vi "IMAQdx_AbsImage_Flea3_v4.2.vi"() -> ()   [LabVIEW 2012]
doc: "Take a single PixelFly exposure and display the result as an intensity graph.This VI illustrates the basics of taking an exposure with the PixelFly camera. Use Ctrl-H to get help on any of the controls\n\nCopyright 2001, The Cooke Corporation."
uses:
  LabVIEW Data V4.10/Shared Libraries/Controls/FileName_Cluster.ctl
  <vilib>/userdefined/High Color/IMAQdx.ctl
  <vilib>/vision/driver/IMAQdx.llb/IMAQdx Acquisition Mode.ctl
  Shared Libraries/Controls/FileInfo_Global.vi
  <vilib>/Analysis/NI_AALBase.lvlib
  <vilib>/vision/driver/NI_Vision_Acquisition_Software.lvlib
panel:
  in  "Interrupt":bool
  out "Buffer Number":u32=4294967294
  out "Frames":i32
  out "Loop":i32=1
  out "Status":string="Running..."
  in  "stop":bool
  in  "Tab Control":enum32{"Setup", "Images", "Hardware status"}(tab)
  in  "Experiment":T1(ring)=enum."Sr"
  in  "Accept parameters from remote system":bool=TRUE
  in  "Bias (Amps)":dbl
  in  "Pinch Coil (Amps)":dbl=520.0
  in  "Expansion time (ms)":dbl=19.0
  in  "Trap min at 0 (MHz)":dbl=2.85
  in  "Detuning (Linewidths)":dbl
  in  "Racetrack (Amps)":dbl=540.0
  in  "Magnification":dbl=0.395
  in  "Image direction":enum16{"XY", "XZ"}(ring)=enum."XZ"
  in  "Imaging technique":enum16{"Absorption", "Fluorescence", "RawImage"}(ring)
  in  "File Parameters":T2={"Data Root"=path "C:/Experiment/Data", "Index"=8, "Instrument"="Flea3_20S4M"} {"Index" format="%04d"}
  in  "Send data to Igor?":bool=TRUE
  out "Command to Igor":string="AutoRunV3(\"MOT_test\",\"C:\\\\Experiment\\\\Data\\\\2012\\\\December\\\\06\\\\Flea3_20S4M_06Dec2012_0007.ibw\") "
  out "Image note":string="Experiment=Sr\nCamera_ID=Flea3\nImageType=Raw\nDataType=Absorption\nImageDirection=XZ\nMagnification=3.950000E-1\nFileNumber=7\n# Current Variables\n# \nplus_zman=-1.791000E+0\nminus_zman=-1.440000E+0\ncompensation=-1.536000E+0\nXshim=1.000000E+1\nYshim=0.000000E+0\nZshim=7.500000E+0\nProbePow=1.200000E+0\ntau=0.000000E+0\ntEnd=0.000000E+0\nDipStart=0.000000E+0\nMOTcurrent=-1.250000E+0\nProbeDet=0.000000E+0\nTOF=5.000000E-4\n# Master Staging List\n# Line\tMarker\tOption\tHalt\t0       4       8      12      16      20    AO\tDelay\t\tPoints\t0\t\t1\t\t2\t\t3\t\t4\t\t5\t\t6\t\t7\t\t8\t\t9\t\t10\t\t11\t\t12\t\t13\t\t14\t\t15\t\tComment\n00\t\tRamp\t0 0 0 0 0 0 0 0 0 0 0 0 1 1 1 1 0 0 0 0 0 0 0 0\t5\t0\tplus_zman\tminus_zman\tcompensation\tMOTcurrent\t0\t0\t0\t0\t0\t0\tProbePow\t0\tXshim\tYshim\tZshim\t0\tblue MOT load\n01\t\tRamp\t0 0 0 0 0 0 0 0 0 0 0 0 1 1 1 1 0 0 0 0 0 0 0 0\t.001\t0\tplus_zman\tminus_zman\tcompensation\tMOTcurrent\t0\t0\t0\t0\t0\t0\tProbePow\t0\tXshim\tYshim\tZshim\t0\tHold\n02\t\tRamp\t0 0 0 0 0 0 0 0 0 0 0 0 1 0 1 1 0 0 0 0 0 0 0 0\t.003\t0\tplus_zman\tminus_zman\tcompensation\tMOTcurrent\t0\t0\t0\t0\t0\t0\tProbePow\t0\tXshim\tYshim\tZshim\t0\tHold\n03\t\tRamp\t0 0 0 0 0 0 0 0 0 0 0 0 1 0 0 0 0 0 0 0 0 0 0 0\tTOF\t0\tplus_zman\tminus_zman\tcompensation\tMOTcurrent\t0\t0\t0\t0\t0\t0\tProbePow\t0\tXshim\tYshim\tZshim\t0\tTOF\n04\t\tRamp\t0 0 0 0 0 0 0 0 0 0 0 0 1 0 0 0 0 0 0 0 0 0 0 0\t.00002\t0\tplus_zman\tminus_zman\tcompensation\tMOTcurrent\t0\t0\t0\t0\t0\t0\tProbePow\t0\tXshim\tYshim\tZshim\t0\tatom img\n05\t\tRamp\t0 0 0 0 0 0 0 0 0 0 0 0 1 1 0 0 0 0 0 0 0 0 0 0\t.0001\t0\tplus_zman\tminus_zman\tcompensation\tMOTcurrent\t0\t0\t0\t0\t0\t0\tProbePow\t0\tXshim\tYshim\tZshim\t0\tatom img\n06\t\tRamp\t0 0 0 0 0 0 0 0 0 0 0 0 1 0 0 0 0 0 0 0 0 0 0 0\t1\t0\tplus_zman\tminus_zman\tcompensation\tMOTcurrent\t0\t0\t0\t0\t0\t0\tProbePow\t0\tXshim\tYshim\tZshim\t0\ttransmit img\n07\t\tRamp\t0 0 0 0 0 0 0 0 0 0 0 0 1 0 0 0 0 0 0 0 0 0 0 0\t.00002\t0\tplus_zman\tminus_zman\tcompensation\tMOTcurrent\t0\t0\t0\t0\t0\t0\tProbePow\t0\tXshim\tYshim\tZshim\t0\tprobe img\n08\t\tRamp\t0 0 0 0 0 0 0 0 0 0 0 0 1 1 0 0 0 0 0 0 0 0 0 0\t.0001\t0\tplus_zman\tminus_zman\tcompensation\tMOTcurrent\t0\t0\t0\t0\t0\t0\tProbePow\t0\tXshim\tYshim\tZshim\t0\tprobe img\n09\t\tRamp\t0 0 0 0 0 0 0 0 0 0 0 0 1 0 0 0 0 0 0 0 0 0 0 0\t0.5\t0\tplus_zman\tminus_zman\tcompensation\tMOTcurrent\t0\t0\t0\t0\t0\t0\tProbePow\t0\tXshim\tYshim\tZshim\t0\ttransmit img\n10\t\tRamp\t0 0 0 0 0 0 0 0 0 0 0 0 1 0 0 0 0 0 0 0 0 0 0 0\t0.5\t0\tplus_zman\tminus_zman\tcompensation\tMOTcurrent\t0\t0\t0\t0\t0\t0\tProbePow\t0\tXshim\tYshim\tZshim\t0\ttransmit img\n11\t\tRamp\t0 0 0 0 0 0 0 0 0 0 0 0 1 0 0 0 0 0 0 0 0 0 0 0\t.00012\t0\tplus_zman\tminus_zman\tcompensation\tMOTcurrent\t0\t0\t0\t0\t0\t0\tProbePow\t0\tXshim\tYshim\tZshim\t0\tbg img\n12\t\tRamp\t0 0 0 0 0 0 0 0 0 0 0 0 1 0 0 0 0 0 0 0 0 0 0 0\t1\t0\tplus_zman\tminus_zman\tcompensation\tMOTcurrent\t0\t0\t0\t0\t0\t0\tProbePow\t0\tXshim\tYshim\tZshim\t0\ttransmit img\n13\t\tRamp\t0 0 0 0 0 0 0 0 0 0 0 0 1 1 1 1 0 0 0 0 0 0 0 0\t.5\t0\tplus_zman\tminus_zman\tcompensation\tMOTcurrent\t0\t0\t0\t0\t0\t0\tProbePow\t0\tXshim\tYshim\tZshim\t0\treset\n14\t\t\t0 0 0 0 0 0 0 0 0 0 0 0 1 1 1 1 0 0 0 0 0 0 0 0\t.1\t0\t\t\t\t\t\t\t\t\t\t\t\t\t\t\t\t\treset\n# Slave Staging List\n# Line\tMarker\tOption\tHalt\t0       4       8      12      16      20    AO\tDelay\t\tPoints\t0\t\t1\t\t2\t\t3\t\t4\t\t5\t\t6\t\t7\t\t8\t\t9\t\t10\t\t11\t\t12\t\t13\t\t14\t\t15\t\tComment\n# SRS List\n# \n#\n# Evaporation\n\nDDS Table\r\n"
  in  "Igor Wave Name":string="Test_Img"
  in  "Save file to archive?":bool=TRUE
  in  "Timeout (ms)":u32=1500
  in  "Gain":dbl
  in  "Shutter speed":dbl=0.03
  in  "Camera Name":T3="Abs XZ"
  out "Timeout":bool=TRUE
  out "Trigger Overrun":bool=TRUE
  in  "Quad [Amps]":dbl=540.0
  in  "Source of File Data":refnum<k21>="\\\\Control\\VariableLibrary\\Instruction String"
  in  "Bits to shift":i32
  in  "Raw image to view":u16(ring) items=["Absorbtion", "Probe", "Background"]
  in  "Update Graphics":bool=TRUE
  out "Raw Image":u16[][](graph)
  out "Processed Image":sgl[][](graph)
  out "Histogram":cluster{"X Values":dbl[], dbl[]}(graph)={"X Values"=[0.296875, 0.890625, 1.484375, 2.078125, 2.671875, 3.265625, 3.859375, 4.453125, 5.046875, 5.640625, 6.234375, 6.828125, 7.421875, 8.015625, 8.609375, 9.203125, 9.796875, 10.390625, 10.984375, 11.578125, 12.171875, 12.765625, 13.359375, 13.953125, 14.546875, 15.140625, 15.734375, 16.328125, 16.921875, 17.515625, 18.109375, 18.703125, 19.296875, 19.890625, 20.484375, 21.078125, 21.671875, 22.265625, 22.859375, 23.453125, 24.046875, 24.640625, 25.234375, 25.828125, 26.421875, 27.015625, 27.609375, 28.203125, 28.796875, 29.390625, 29.984375, 30.578125, 31.171875, 31.765625, 32.359375, 32.953125, 33.546875, 34.140625, 34.734375, 35.328125, 35.921875, 36.515625, 37.109375, 37.703125], [5.35923388091367, 4.928319024503722, -inf, 5.005013113795492, -inf, 5.057559608844285, 5.110747912804027, -inf, 5.127593914375556, -inf, 5.149274550965593, 5.147097910277923, -inf, 5.125201405320576, -inf, 5.104084041079007, 5.05411873464641, -inf, 5.006016539554038, -inf, 4.958396630923071, 4.877883672326599, -inf, 4.808224481096161, -inf, 4.725029085721709, 4.615550274725666, -inf, 4.51079961442428, -inf, 4.383599959933904, -inf, 4.2468677218991155, 4.1075830311913215, -inf, 3.9644482079166607, -inf, 3.801952234854282, 3.637189422148762, -inf, 3.443888546777372, -inf, 3.2467447097238415, 3.0729847446279304, -inf, 2.8555191556678, -inf, 2.597695185925512, 2.3096301674258988, -inf, 2.089905111439398, -inf, 1.8260748027008264, 1.6127838567197355, -inf, 1.3222192947339193, -inf, 0.9030899869919435, 0.6989700043360189, -inf, 0.0, -inf, -inf, 0.3010299956639812]}
  out "Images":u16[][][](array[numeric])
  out "Camera Error":errorcluster={"status"=FALSE, "code"=-1074360293, "source"="IMAQdx Get Image.vi"}
  out "DDE Error":errorcluster={"status"=FALSE, "code"=0, "source"="DDE Close: No Error"}
  out "Status Array":T4(array[cluster])=[{"AcquisitionInProgress"=FALSE, "BufferCount"=1447, "LastBufferNumber"=1446, "LostBufferCount"=0}, {"AcquisitionInProgress"=TRUE, "BufferCount"=0, "LastBufferNumber"=4294967292, "LostBufferCount"=0}, {"AcquisitionInProgress"=TRUE, "BufferCount"=0, "LastBufferNumber"=4294967292, "LostBufferCount"=0}, {"AcquisitionInProgress"=TRUE, "BufferCount"=0, "LastBufferNumber"=4294967292, "LostBufferCount"=0}, {"AcquisitionInProgress"=TRUE, "BufferCount"=0, "LastBufferNumber"=4294967292, "LostBufferCount"=0}, {"AcquisitionInProgress"=TRUE, "BufferCount"=0, "LastBufferNumber"=4294967292, "LostBufferCount"=0}, {"AcquisitionInProgress"=TRUE, "BufferCount"=0, "LastBufferNumber"=4294967292, "LostBufferCount"=0}, {"AcquisitionInProgress"=TRUE, "BufferCount"=0, "LastBufferNumber"=4294967292, "LostBufferCount"=0}, {"AcquisitionInProgress"=TRUE, "BufferCount"=0, "LastBufferNumber"=4294967292, "LostBufferCount"=0}, {"AcquisitionInProgress"=TRUE, "BufferCount"=0, "LastBufferNumber"=4294967292, "LostBufferCount"=0}, {"AcquisitionInProgress"=TRUE, "BufferCount"=0, "LastBufferNumber"=4294967292, "LostBufferCount"=0}, {"AcquisitionInProgress"=TRUE, "BufferCount"=0, "LastBufferNumber"=4294967292, "LostBufferCount"=0}, {"AcquisitionInProgress"=TRUE, "BufferCount"=0, "LastBufferNumber"=4294967292, "LostBufferCount"=0}, {"AcquisitionInProgress"=TRUE, "BufferCount"=0, "LastBufferNumber"=4294967292, "LostBufferCount"=0}, {"AcquisitionInProgress"=TRUE, "BufferCount"=0, "LastBufferNumber"=4294967292, "LostBufferCount"=0}, {"AcquisitionInProgress"=TRUE, "BufferCount"=0, "LastBufferNumber"=4294967292, "LostBufferCount"=0}, {"AcquisitionInProgress"=TRUE, "BufferCount"=1, "LastBufferNumber"=0, "LostBufferCount"=0}, {"AcquisitionInProgress"=TRUE, "BufferCount"=2, "LastBufferNumber"=1, "LostBufferCount"=0}, {"AcquisitionInProgress"=TRUE, "BufferCount"=3, "LastBufferNumber"=2, "LostBufferCount"=0}]
  # "Flea3 Image Acquisition v4.2"
  # "Experimental Paramaters"
  # "Cam0 is XZ, Cam1 is XY"
  # "RbYb: set to 0."
  # "The only get set on 1st run.\nUse  a Gain of 10:\n* Seems to give a readout error of 1 bit.\n* Know intensity calibration"
  # "In both techniques 3 images\nare aquired, but in Fluorescense\nthe 3rd is discarded"
  # "Sr: .395  is XZ\n     ----- is XY"
  # "Obsolete: (now done with network variables)\nWhen paramaters are accepted from a remote system a DataSockets server\nmust be running on this machine (in start menu in National Instruments folder)"
  # "Camera configuration"
  # "File configuration"
  # "When the gain is 10 :  742 counts = Isat with 100 us pulse.  This is fine and\nis the point of highest SNR.  Linearized in software."
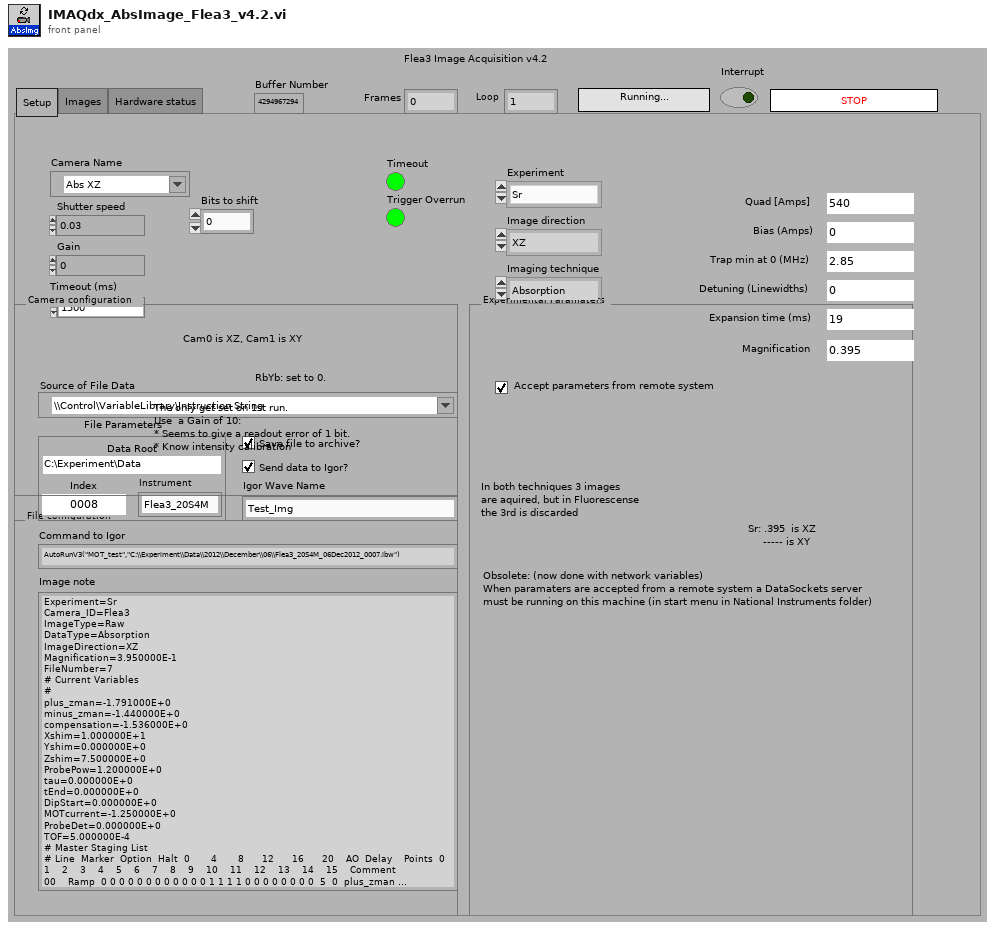
[diagram p1: front panel]
types:
  T1 = enum16{"Rubidium I", "Rubidium II", "RbLi", "RbYb", "Sr"}
  T2 = typedef "FileName_Cluster.ctl" = cluster{"Data Root":path, "Index":u32, "Instrument":string}
  T3 = typedef "IMAQdx.ctl" = refnum<k21>
  T4 = cluster{"AcquisitionInProgress":bool, "BufferCount":u32, "LastBufferNumber":u32, "LostBufferCount":u32}[]
  T5 = typedef "NI_Vision_Acquisition_Software.lvlib/IMAQdx Acquisition Mode.ctl" = enum32{"One Shot", "Continuous"}
  T6 = typedef "Image Type" = u32
  T7 = typedef "IMAQ Image.ctl" = refnum<image>
  T8 = cluster{"AcquisitionInProgress":bool, "BufferCount":u32, "LastBufferNumber":u32, "LostBufferCount":u32}
  T9 = cluster{"X Values":dbl[], "Histogram: h(x)":i32[]}
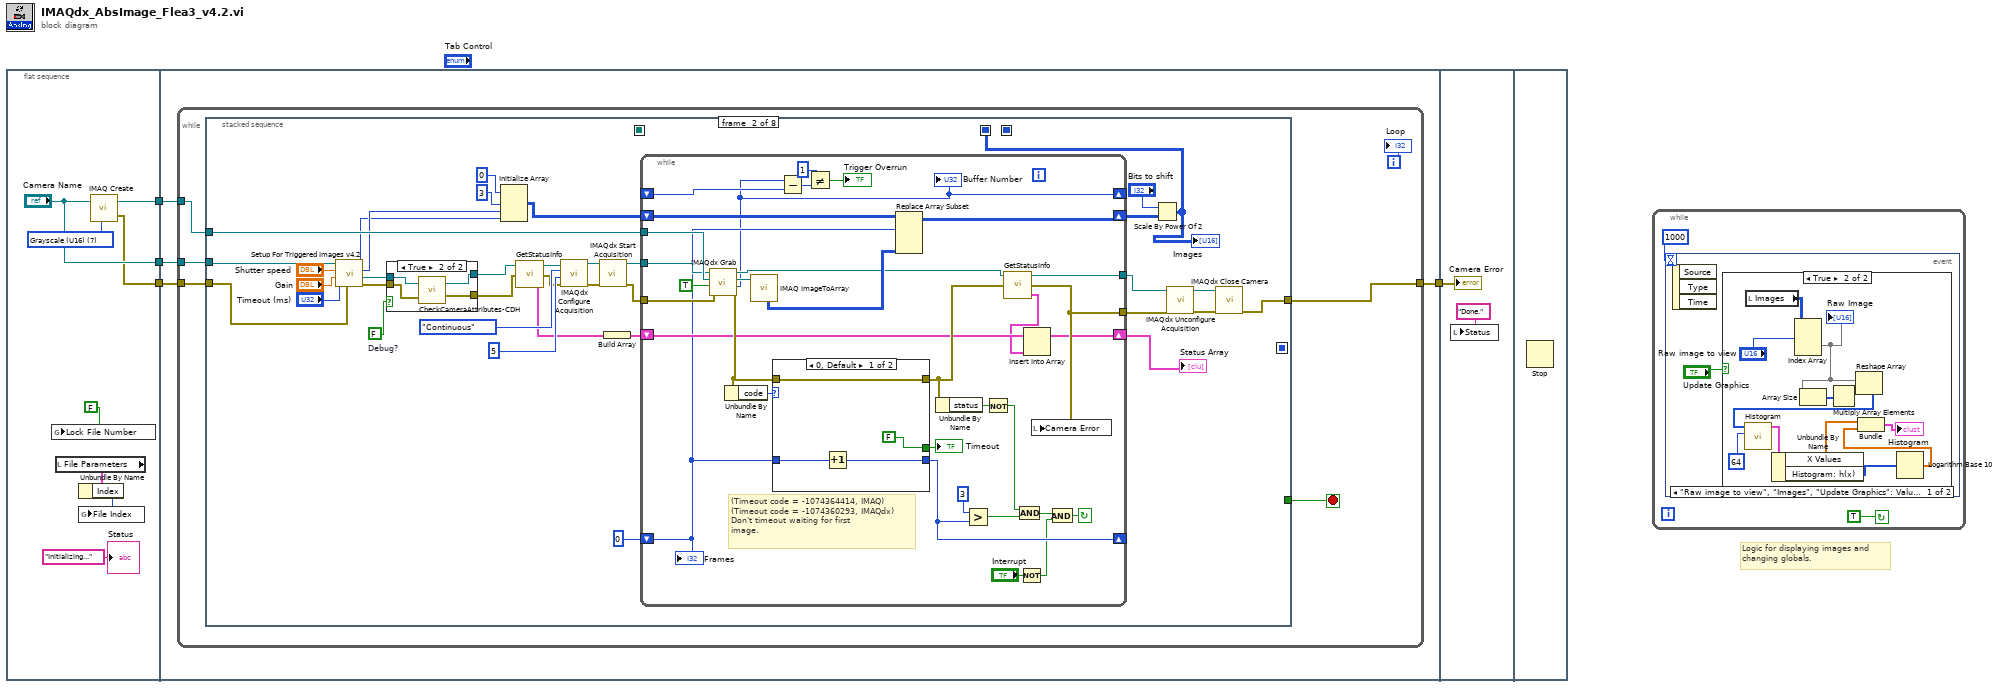
[diagram p0: block diagram]
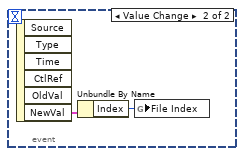
[diagram p3: hidden frame]
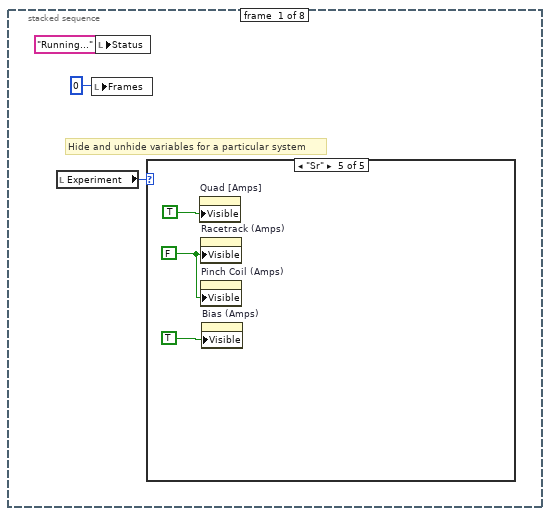
[diagram p4: hidden frame]
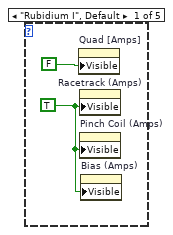
[diagram p5: hidden frame]
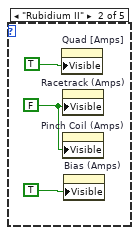
[diagram p6: hidden frame]
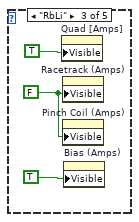
[diagram p7: hidden frame]
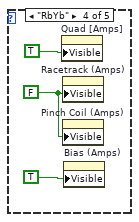
[diagram p8: hidden frame]
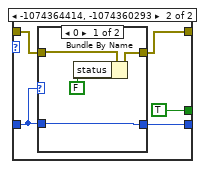
[diagram p10: hidden frame]
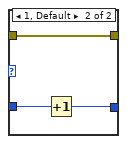
[diagram p11: hidden frame]
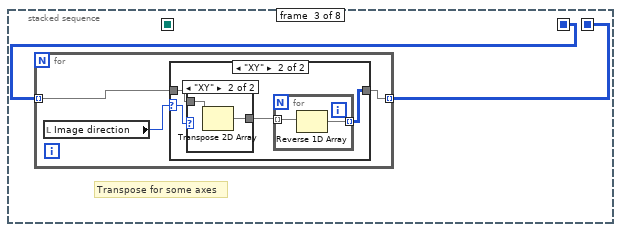
[diagram p12: hidden frame]
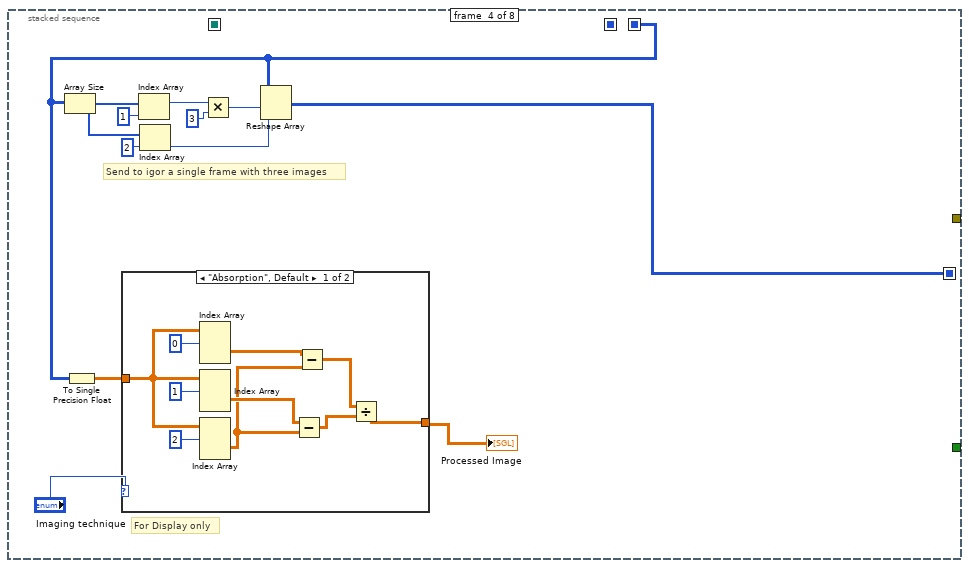
[diagram p15: hidden frame]
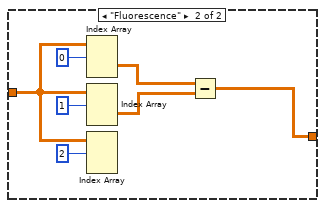
[diagram p16: hidden frame]
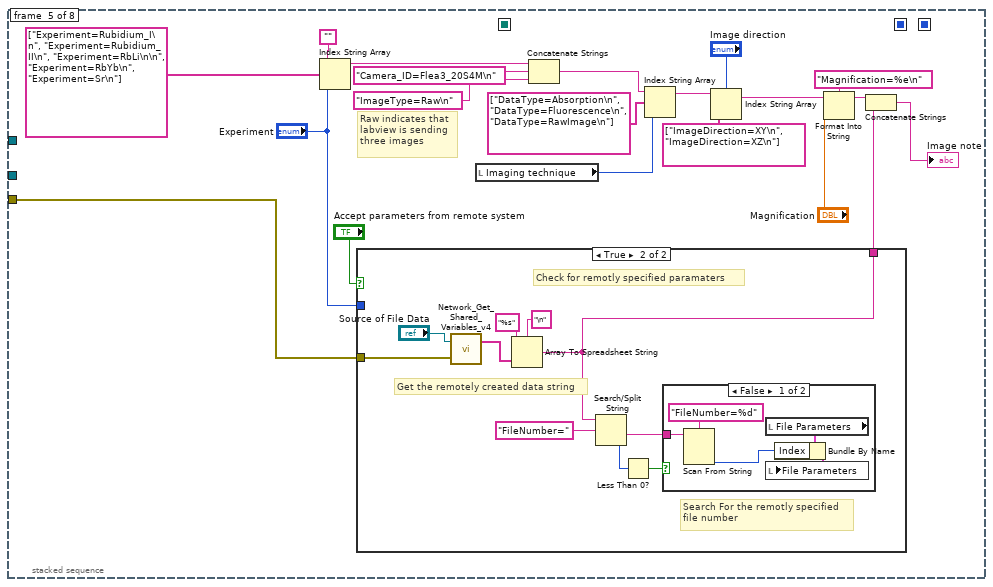
[diagram p17: hidden frame]
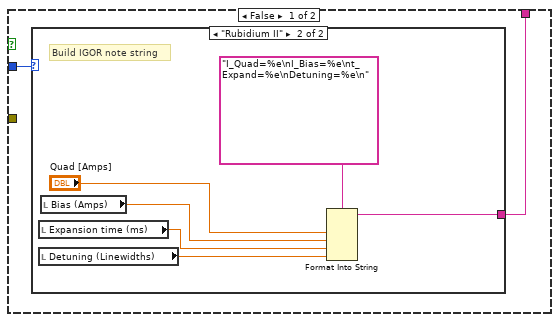
[diagram p18: hidden frame]
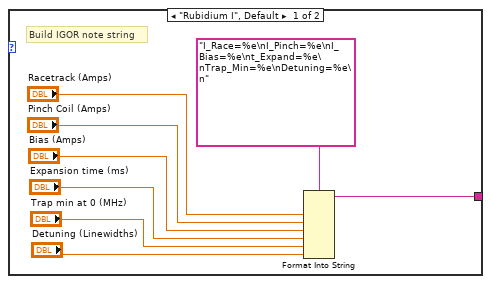
[diagram p19: hidden frame]
diagram:
  # "Logic for displaying images and\nchanging globals."
  n1 = flat-sequence {
    tunnel: [w8] -> w4
    tunnel: ["Camera Name"] -> w3
    tunnel: [w6] -> w2
    tunnel: w3 -> [w16]
    tunnel: w4 -> [w15]
    tunnel: w2 -> [w14]
    tunnel: [w13] -> w1
    tunnel: w1 -> [w258]
    frame #0 {
      w5 = T6 7 items=["Grayscale (U8)", "Grayscale (I16)", "Grayscale (SGL)", "Complex (CSG)", "RGB (U32)", "HSL (U32)", "RGB (U64)", "Grayscale (U16)"] ("Image Type")
      n2 = global write "FileInfo_Global.vi" "Lock File Number"(FALSE) -> ()
      n3 = local read "File Parameters"() -> (w9:T2)
      n4 = Unbundle By Name(w9) -> ("Index"=w10:u32)
      n5 = global write "FileInfo_Global.vi" "File Index"(w10) -> ()
      n6 = call "IMAQ Create"("Image Name"="Camera Name", "Image Type"=w5) -> ("New Image"=w8:T7, "error out"=w6:errorcluster)  [unwired: 2 in, 1 out]
      "Status" <- "Initializing..."
    }
    frame #1 {
      n7 = while {
        tunnel: w16 -> [w19]
        tunnel: w15 -> [w20]
        tunnel: w14 -> [w18]
        tunnel: [w17] -> w13
        i -> [w22]
        stop <- w21 stop-if-true
        n8 = stacked-sequence {
          seq-local: [_ _ _ w155 _ _ _ _] -> [_ _ _ _ _ w230 _ _]
          seq-local: [_ _ _ _ _ w226 _ _] -> [_ _ _ _ _ _ _ w240]
          seq-local: [_ w60 _ _ _ _ _ _] -> [_ _ w132 _ _ _ _ _]
          seq-local: [_ _ w131 _ _ _ _ _] -> [_ _ _ w146 _ _ _ _]
          tunnel: [_ _ _ _ _ _ _ "stop"] -> w21
          tunnel: w18 -> [_ w66 _ _ w182 _ _ _]
          tunnel: w19 -> [_ w67 _ _ _ _ _ _]
          tunnel: w20 -> [_ w75 _ _ _ _ _ _]
          tunnel: [_ w65 _ _ _ _ _ _] -> w17
          frame #0 {
            # "Hide and unhide variables for a particular system"
            n9 = local read "Experiment"() -> (w23:T1)
            n10 = local write "Frames"(0) -> ()
            n11 = local write "Status"("Running...") -> ()
            n12 = case shown="\"Sr\"" w23 {
              frame "Rubidium I", Default {
                w26 = TRUE
                n13 = property on="Quad [Amps]" class="DigNum (strict)"("Visible"=FALSE) -> ()  [unwired: 2 in, 2 out]
                n14 = property on="Racetrack (Amps)" class="DigNum (strict)"("Visible"=w26) -> ()  [unwired: 2 in, 2 out]
                n15 = property on="Pinch Coil (Amps)" class="DigNum (strict)"("Visible"=w26) -> ()  [unwired: 2 in, 2 out]
                n16 = property on="Bias (Amps)" class="DigNum (strict)"("Visible"=w26) -> ()  [unwired: 2 in, 2 out]
              }
              frame "Rubidium II" {
                w29 = FALSE
                n17 = property on="Quad [Amps]" class="DigNum (strict)"("Visible"=TRUE) -> ()  [unwired: 2 in, 2 out]
                n18 = property on="Racetrack (Amps)" class="DigNum (strict)"("Visible"=w29) -> ()  [unwired: 2 in, 2 out]
                n19 = property on="Pinch Coil (Amps)" class="DigNum (strict)"("Visible"=w29) -> ()  [unwired: 2 in, 2 out]
                n20 = property on="Bias (Amps)" class="DigNum (strict)"("Visible"=TRUE) -> ()  [unwired: 2 in, 2 out]
              }
              frame "RbLi" {
                w32 = FALSE
                n21 = property on="Quad [Amps]" class="DigNum (strict)"("Visible"=TRUE) -> ()  [unwired: 2 in, 2 out]
                n22 = property on="Racetrack (Amps)" class="DigNum (strict)"("Visible"=w32) -> ()  [unwired: 2 in, 2 out]
                n23 = property on="Pinch Coil (Amps)" class="DigNum (strict)"("Visible"=w32) -> ()  [unwired: 2 in, 2 out]
                n24 = property on="Bias (Amps)" class="DigNum (strict)"("Visible"=TRUE) -> ()  [unwired: 2 in, 2 out]
              }
              frame "RbYb" {
                w35 = FALSE
                n25 = property on="Quad [Amps]" class="DigNum (strict)"("Visible"=TRUE) -> ()  [unwired: 2 in, 2 out]
                n26 = property on="Racetrack (Amps)" class="DigNum (strict)"("Visible"=w35) -> ()  [unwired: 2 in, 2 out]
                n27 = property on="Pinch Coil (Amps)" class="DigNum (strict)"("Visible"=w35) -> ()  [unwired: 2 in, 2 out]
                n28 = property on="Bias (Amps)" class="DigNum (strict)"("Visible"=TRUE) -> ()  [unwired: 2 in, 2 out]
              }
              frame "Sr" {
                w38 = FALSE
                n29 = property on="Quad [Amps]" class="DigNum (strict)"("Visible"=TRUE) -> ()  [unwired: 2 in, 2 out]
                n30 = property on="Racetrack (Amps)" class="DigNum (strict)"("Visible"=w38) -> ()  [unwired: 2 in, 2 out]
                n31 = property on="Pinch Coil (Amps)" class="DigNum (strict)"("Visible"=w38) -> ()  [unwired: 2 in, 2 out]
                n32 = property on="Bias (Amps)" class="DigNum (strict)"("Visible"=TRUE) -> ()  [unwired: 2 in, 2 out]
              }
            }
          }
          frame #1 {
            w53 = FALSE  # Debug?
            n33 = call "Setup For Triggered Images v4.2.vi"("error in"=w66, "Timeout (ms)"="Timeout (ms)", "Gain"="Gain", "Shutter speed"="Shutter speed", "Camera Name"=w67) -> ("Error out"=w54:errorcluster, "Session Out"=w55:T3, "Height"=w64:u32, "Width"=w63:u32)
            n34 = case shown="True" w53 {
              tunnel: [w76 w81] -> w49
              tunnel: [w77 w80] -> w46
              tunnel: w55 -> [w76 w79]
              tunnel: w54 -> [w77 w78]
              frame False {
              }
              frame True {
                n35 = call "CheckCameraAttributes-CDH.vi"("error in"=w78, "Camera Name"=w79) -> ("error out"=w80:errorcluster, "Session Out"=w81:T3)
              }
            }
            n36 = Initialize Array(u16 0, 3, w64, w63) -> (w71:u16[][][])
            n37 = call "GetStatusInfo.vi"("error in"=w46, "Camera In"=w49) -> ("Status Info"=w45:T8, "error out"=w47:errorcluster, "Camera Out"=w48:T3)  [unwired: 1 in]
            n38 = call <vilib>:"IMAQdx Configure Acquisition.vi"("error in"=w47, "Number of Buffers"=u32 5, "Continuous?"=IMAQdx_Acquisition_Mode."Continuous", "Session In"=w48) -> ("error out"=w56:errorcluster, "Session Out"=w57:T3)  [unwired: 6 in]
            n39 = call <vilib>:"IMAQdx Start Acquisition.vi"("error in"=w56, "Session In"=w57) -> ("error out"=w50:errorcluster, "Session Out"=w51:T3)  [unwired: 8 out]
            n40 = Build Array(w45) -> (w52:T4)
            n41 = while {
              tunnel: w75 -> [w104]
              shift-right: [w82] -> _
              shift-left: _ -> [w109]
              tunnel: [w90] -> w43
              tunnel: w50 -> [w102]
              tunnel: [w87] -> w41
              shift-right: [w97] -> _
              shift-left: 0 -> [w84]
              shift-right: [w105] -> w61
              shift-left: w71 -> [w106]
              tunnel: w51 -> [w103]
              shift-right: [w85] -> w44
              shift-left: w52 -> [w86]
              stop <- w93 continue-if-true
              # "(Timeout code = -1074364414, IMAQ)\n(Timeout code = -1074360293, IMAQdx)\nDon't timeout waiting for first\nimage."
              n42 = call <vilib>:"IMAQdx Grab.vi"("error in"=w102, "Wait for Next Buffer? (Yes)"=TRUE, "Image In"=w104, "Session In"=w103) -> ("error out"=w101:errorcluster, "Buffer Number Out"=w82:u32, "Image Out"=w96:T7, "Session Out"=w89:T3)  [unwired: 4 out]
              "Buffer Number" <- w82
              n43 = Unbundle By Name(w101) -> ("code"=w113:i32)
              n44 = call "IMAQ ImageToArray"("Image"=w96) -> ("Image Pixels (U16)"=w95:u16[][])  [unwired: 2 in, 5 out]
              n45 = case shown="0, Default" w113 {
                tunnel: w101 -> [w118 w122]
                tunnel: [w118 w121] -> w88
                tunnel: [FALSE TRUE] -> w114
                tunnel: w84 -> [w116 w120]
                tunnel: [w115 w119] -> w97
                frame 0, Default {
                  n46 = Increment(x=w116) -> (x+1=w115:i32)
                }
                frame -1074364414, -1074360293 {
                  n47 = case shown="0" w120 {
                    tunnel: [w124 w130] -> w121
                    tunnel: w122 -> [w126 w130]
                    tunnel: w120 -> [w125 w129]
                    tunnel: [w125 w128] -> w119
                    frame 0 {
                      n48 = Bundle By Name(cluster=w126, "status"=FALSE) -> (w124:errorcluster)
                    }
                    frame 1, Default {
                      n49 = Increment(x=w129) -> (x+1=w128:i32)
                    }
                  }
                }
              }
              "Timeout" <- w114
              n50 = Subtract(x=w82, y=w109) -> (x-y=w110:u32)
              n51 = Not Equal?(x=u32 1, y=w110) -> (x != y?=→"Trigger Overrun":bool)
              n52 = Replace Array Subset(array=w106, new element=w95, index (dim 0)=w84) -> (w105:u16[][][])  [unwired: 2 in]
              n53 = Unbundle By Name(w88) -> ("status"=w108:bool)
              n54 = Greater?(x=3, y=w97) -> (0:w98:bool)
              n55 = Not(x=w108) -> (.not. x?=w107:bool)
              n56 = call "GetStatusInfo.vi"("error in"=w88, "Camera In"=w89) -> ("Status Info"=w83:T8, "error out"=w87:errorcluster, "Camera Out"=w90:T3)  [unwired: 1 in]
              n57 = And(x=w107, y=w98) -> (x .and. y?=w94:bool)
              n58 = Not(x="Interrupt") -> (.not. x?=w91:bool)
              n59 = Insert Into Array(array=w86, new element=w83) -> (w85:T4)  [unwired: 1 in]
              n60 = local write "Camera Error"(w87) -> ()
              n61 = And(x=w94, y=w91) -> (x .and. y?=w93:bool)
              "Frames" <- w84
            }
            "Status Array" <- w44
            n62 = Scale By Power Of 2(n="Bits to shift", x=w61) -> (x*2^n=w60:u16[][][])
            "Images" <- w60
            n63 = call <vilib>:"IMAQdx Unconfigure Acquisition.vi"("error in"=w41, "Session In"=w43) -> ("error out"=w40:errorcluster, "Session Out"=w42:T3)  [unwired: 8 in]
            n64 = call <vilib>:"IMAQdx Close Camera.vi"("error in"=w40, "Session In"=w42) -> ("error out"=w65:errorcluster)  [unwired: 9 out]
          }
          frame #2 {
            # "Transpose for some axes"
            n65 = for {
              tunnel: w132 -> [w134] mode=indexing
              tunnel: [w133] -> w131 mode=indexing
              n66 = local read "Image direction"() -> (w135:enum16{"XY", "XZ"})
              n67 = case shown="\"XY\"" w135 {
                selector: w135 -> [_ w137]
                tunnel: w134 -> [w136 w139]
                tunnel: [w136 w140] -> w133
                frame Default {
                }
                frame "XY" {
                  n68 = case shown="\"XY\"" w137 {
                    tunnel: w139 -> [w141 w143]
                    tunnel: [w141 w142] -> w138
                    frame Default {
                    }
                    frame "XY" {
                      n69 = Transpose 2D Array(2D array=w143) -> (transposed array=w142:u16[][])
                    }
                  }
                  n70 = for {
                    tunnel: w138 -> [w145] mode=indexing
                    tunnel: [w144] -> w140 mode=indexing
                    n71 = Reverse 1D Array(array=w145) -> (reversed array=w144:u16[])
                  }
                }
              }
            }
          }
          frame #3 {
            # "Send to igor a single frame with three images"
            # "For Display only"
            n72 = Array Size(array=w146) -> (size(s)=w151:i32[])
            n73 = To Single Precision Float(number=w146) -> (single precision float=w152:sgl[][][])
            n74 = case shown="\"Absorption\", Default" "Imaging technique" {
              tunnel: [w164 w170] -> w156
              tunnel: w152 -> [w163 w171]
              frame "Absorption", Default {
                n75 = Index Array(array=w163, index (dim 0)=0 ("Number of buffers")) -> (element=w162:sgl[][])  [unwired: 2 in]
                n76 = Index Array(array=w163, index (dim 0)=1 ("Number of buffers")) -> (element=w161:sgl[][])  [unwired: 2 in]
                n77 = Index Array(array=w163, index (dim 0)=2 ("Number of buffers")) -> (element=w160:sgl[][])  [unwired: 2 in]
                n78 = Subtract(x=w161, y=w160) -> (x-y=w159:sgl[][])
                n79 = Subtract(x=w162, y=w160) -> (x-y=w158:sgl[][])
                n80 = Divide(x=w158, y=w159) -> (x/y=w164:sgl[][])
              }
              frame "Fluorescence" {
                n81 = Index Array(array=w171, index (dim 0)=0 ("Number of buffers")) -> (element=w169:sgl[][])  [unwired: 2 in]
                n82 = Index Array(array=w171, index (dim 0)=1 ("Number of buffers")) -> (element=w168:sgl[][])  [unwired: 2 in]
                n83 = Index Array(array=w171, index (dim 0)=2 ("Number of buffers")) -> ()  [unwired: 2 in, 1 out]
                n84 = Subtract(x=w169, y=w168) -> (x-y=w170:sgl[][])
              }
            }
            "Processed Image" <- w156
            n85 = Index Array(array=w151, index=1 ("Number of buffers")) -> (element=w148:i32)
            n86 = Index Array(array=w151, index=2 ("Number of buffers")) -> (element=w147:i32)
            n87 = Multiply(x=w148, y=3 ("Number of buffers")) -> (x*y=w153:i32)
            n88 = Reshape Array(w146, w153, w147) -> (w155:u16[][])
          }
          frame #4 {
            # "Raw indicates that\nlabview is sending\nthree images"
            n89 = Index String Array(1:"Experiment", 2:string[] ["Experiment=Rubidium_I\n", "Experiment=Rubidium_II\n", "Experiment=RbLi\n\n", "Experiment=RbYb\n", "Experiment=Sr\n"], 3:"") -> (0:w179:string)
            n90 = case shown="True" "Accept parameters from remote system" {
              tunnel: w182 -> [_ w220]
              tunnel: [w196 w212] -> w186
              tunnel: "Experiment" -> [w195 _]
              frame False {
                n91 = case shown="\"Rubidium II\"" w195 {
                  tunnel: [w197 w208] -> w196
                  frame "Rubidium I", Default {
                    # "Build IGOR note string"
                    n92 = Format Into String(format string="I_Race=%e\nI_Pinch=%e\nI_Bias=%e\nt_Expand=%e\nTrap_Min=%e\nDetuning=%e\n", "Racetrack (Amps)", "Pinch Coil (Amps)", "Bias (Amps)", "Expansion time (ms)", "Trap min at 0 (MHz)", "Detuning (Linewidths)") -> (resulting string=w197:string)  [unwired: 2 in, 1 out]
                  }
                  frame "Rubidium II" {
                    # "Build IGOR note string"
                    n93 = local read "Expansion time (ms)"() -> (w206:dbl)
                    n94 = local read "Detuning (Linewidths)"() -> (w205:dbl)
                    n95 = local read "Bias (Amps)"() -> (w207:dbl)
                    n96 = Format Into String(format string="I_Quad=%e\nI_Bias=%e\nt_Expand=%e\nDetuning=%e\n", "Quad [Amps]", w207, w206, w205) -> (resulting string=w208:string)  [unwired: 2 in, 1 out]
                  }
                }
              }
              frame True {
                # "Check for remotly specified paramaters"
                # "Get the remotely created data string"
                # "Search For the remotly specified\nfile number"
                n97 = call "Network_Get_Shared_Variables_v4.vi"("error in (no error)"=w220, "Source of Data"="Source of File Data") -> ("Igor Instruction String"=w219:string[])  [unwired: 1 out]
                n98 = Array To Spreadsheet String(delimiter (Tab)="\n", array=w219, 3:"%s") -> (spreadsheet string=w212:string)
                n99 = Search/Split String(string=w212, search string/char (-)="FileNumber=") -> (match + rest of string=w215:string, offset of match=w214:i32)  [unwired: 2 out]
                n100 = Less Than 0?(x=w214) -> (x < 0?=w213:bool)
                n101 = case shown="False" w213 {
                  tunnel: w215 -> [w225 _]
                  frame False {
                    n102 = Scan From String(format string="FileNumber=%d", input string=w225) -> (output 1=w221:i32)  [unwired: 2 in, 4 out]
                    n103 = local read "File Parameters"() -> (w223:T2)
                    n104 = Bundle By Name(cluster=w223, "Index"=w221) -> (w222:T2)
                    n105 = local write "File Parameters"(w222) -> ()
                  }
                  frame True {
                  }
                }
              }
            }
            n106 = local read "Imaging technique"() -> (w191:enum16{"Absorption", "Fluorescence", "RawImage"})
            n107 = Concatenate Strings(w179, "Camera_ID=Flea3_20S4M\n", "ImageType=Raw\n") -> (w180:string)
            n108 = Index String Array(1:w191, 2:string[] ["DataType=Absorption\n", "DataType=Fluorescence\n", "DataType=RawImage\n"], 3:w180) -> (0:w192:string)
            n109 = Index String Array(1:"Image direction", 2:string[] ["ImageDirection=XY\n", "ImageDirection=XZ\n"], 3:w192) -> (0:w194:string)
            n110 = Format Into String(format string="Magnification=%e\n", initial string=w194, "Magnification") -> (resulting string=w188:string)  [unwired: 1 in, 1 out]
            n111 = Concatenate Strings(w188, w186) -> (→"Image note":string)
          }
          frame #5 {
            # "Save the file as an igor binary"
            n112 = call "MakeFileName_NIST.vi"("File Parameters"="File Parameters", "Save permanent file?"="Save file to archive?") -> ("New file parameters."=w232:T2, "Path to File"=w234:path, "path"=w233:path)
            n113 = local write "File Parameters"(w232) -> ()
            n114 = call "RecursiveMakeDirectory.vi"("Directory to create"=w233) -> ("error out"=w236:errorcluster)  [unwired: 1 in, 1 out]
            n115 = local read "Image note"() -> (w229:string)
            n116 = Delete(path (use dialog)=w234, error in=w236) -> (deleted path=w227:path)  [unwired: 5 out]
            n117 = call "2D INT16 to Igor Binary File.vi"("Wave Data (I16)"=w230, "Wave Note (\"\")"=w229, "WaveName"="Igor Wave Name", "Path (default: dialog)"=w227) -> ("Path chosen"=w226:path)
          }
          frame #6 {
            # "Be sure the file is written"
            n118 = Wait (ms)(milliseconds to wait=u32 1000) -> ()  [unwired: 1 out]
          }
          frame #7 {
            n119 = case shown="True" "Send data to Igor?" {
              tunnel: w240 -> [_ w249]
              tunnel: ["" w248] -> w239
              frame False {
              }
              frame True {
                # "Tell Igor what file to open"
                n120 = Path To String(path=w249) -> (string=w246:string)
                n121 = call <vilib>:"DDE Open Conversation.vi"("topic"="Igor", "service"="Igor") -> ("error out"=w253:errorcluster, "conversation refnum"=w251:u32)  [unwired: 1 in, 5 out]
                n122 = Search and Replace String(replace all?=TRUE, input string=w246, search string="\\", replace string="\\\\") -> (result string=w247:string)  [unwired: 1 in, 6 out]
                n123 = Format Into String(format string="AutoRunV3(\"Mot_T_Sr_88\",\"%s\") ", w247) -> (resulting string=w248:string)  [unwired: 2 in, 1 out]
                n124 = call <vilib>:"DDE Execute.vi"("error in (no error)"=w253, "command"=w248, "conversation refnum in"=w251) -> ("error out"=w252:errorcluster, "conversation refnum out"=w250:u32)  [unwired: 5 out]
                n125 = call <vilib>:"DDE Close Conversation.vi"("error in (no error)"=w252, "conversation refnum"=w250) -> ("error out"=→"DDE Error":errorcluster)  [unwired: 7 out]
              }
            }
            "Command to Igor" <- w239
          }
        }
        "Loop" <- w22
      }
    }
    frame #2 {
      n126 = local write "Status"("Done.") -> ()
      "Camera Error" <- w258
    }
    frame #3 {
      n127 = Stop() -> ()  [unwired: 1 out]
    }
  }
  n128 = while {
    stop <- TRUE continue-if-true
    n129 = event shown="[0] \"Raw image to view\", \"Images\", \"Update Graphics\": Value Change;  Timeout" {
      selector: _ -> [_ _]
      dyn-events: _ -> [_ _]
      timeout: 1000 -> [_ _]
      event "Raw image to view", "Images", "Update Graphics": Value Change; Timeout {
        n130 = event-data() -> ()  [unwired: 4 out]
        n131 = case shown="True" "Update Graphics" {
          frame False {
          }
          frame True {
            n132 = local read "Images"() -> (w274:u16[][][])
            n133 = Index Array(array=w274, index (dim 0)="Raw image to view") -> (element=w272:u16[][])  [unwired: 2 in]
            "Raw Image" <- w272
            n134 = Array Size(array=w272) -> (size(s)=w271:i32[])
            n135 = Multiply Array Elements(1:w271) -> (0:w270:i32)
            n136 = Reshape Array(w272, w270) -> (w268:u16[])
            n137 = call <vilib>:"Histogram.vi"("intervals"=64, "X"=w268) -> ("Histogram Graph"=w267:T9)  [unwired: 9 out]
            n138 = Unbundle By Name(w267) -> ("X Values"=w265:dbl[], "Histogram: h(x)"=w266:i32[])
            n139 = Logarithm Base 10(1:w266) -> (0:w264:dbl[])
            n140 = Bundle("X Values"=w265, w264) -> (→"Histogram":cluster{"X Values":dbl[], dbl[]})  [unwired: 1 out]
          }
        }
      }
      event Value Change {
        n141 = event-data() -> ("NewVal"=w275:T2)  [unwired: 6 out]
        n142 = Unbundle By Name(w275) -> ("Index"=w276:u32)
        n143 = global write "FileInfo_Global.vi" "File Index"(w276) -> ()
      }
    }
  }
